vi "MartinsDCposition.vi"() -> ()   [LabVIEW 2011]
uses:
  Sub VIs/Trap cluster.ctl
  <vilib>/Utility/inputDevices.llb/closeKeyboard.vi
  <vilib>/Utility/inputDevices.llb/keyboardAcquire.vi
  <vilib>/vision/driver/NI_Vision_Acquisition_Software.lvlib
panel:
  in  "e_desired":sgl=0.5
  in  "Apply Corrections":bool
  in  "View Licence":bool
  in  "ok":bool caption="Mark the center of \nthe spot using the \nzoom and the point\ntool, then click this \nbutton"
  in  "Stop program":bool
  in  "Updating trap cluster":bool
  out "Camera enabled":bool
  out "SLM enabled":bool
  in  "Run calibration":bool
  in  "Hologram generation":cluster{"Method":i32, "Iterations":i32}={"Method"=0, "Iterations"=10} {"Method" items=["Lenses & Gratings (3D)", " Gerchberg-Saxton (3D)", "Gerchberg-Saxton FFT (2D)"]}
  in  "Display hologram\nand computed \nimage plane":bool=TRUE
  in  "ROI":T1={"Global Rectangle"=[568, 568, 719, 569], "Contours"=[{"Contour Type"=0, "ROI Type"=1, "Points"=[568, 568]}, {"Contour Type"=0, "ROI Type"=1, "Points"=[642, 568]}, {"Contour Type"=0, "ROI Type"=1, "Points"=[718, 568]}]}
  out "Image":T2(plugin-control)
  in  "y":dbl=100.0 min=1e-22
  in  "Show image":bool=TRUE
  in  "ROI size":dbl=2.0 min=2.0 step=2.0
  in  "Tab Control":enum32{"Normal", "Grid"}(tab)=enum."Grid"
  in  "Z":dbl[](array[numeric])=[0.0, 0.0, 0.0]
  in  "I":dbl[](array[numeric])=[10.0, 10.0, 10.0]
  out "#":i32[](array[numeric])=[0, 1, 2]
  in  "G":bool[](array[boolean])=[FALSE, FALSE, FALSE]
  in  "Spots y":i32=3
  in  "Grid spacing":i32=35
  in  "Spots x":i32=3
  in  "separation step":i32=1
  in  "max separation":i32=40
  in  "min separation":i32=30
  in  "Measure":bool
  in  "#images":i32=1
  out "Step number":i32
  in  "Move one spot":bool
  out "Calculated image plane":dbl[][](graph)
  out "Current trap pos":T3={"X (IMAQ)"=[555.0, 642.5, 730.0, 555.0, 642.5, 730.0, 555.0, 642.5, 730.0], "Y (IMAQ)"=[555.0, 555.0, 555.0, 642.5, 642.5, 642.5, 730.0, 730.0, 730.0], "Z"=[0.0, 0.0, 0.0, 0.0, 0.0, 0.0, 0.0, 0.0, 0.0], "Amplitudes"=[1.0, 1.0, 1.0, 1.0, 1.0, 1.0, 1.0, 1.0, 1.0], "Trap number"=[0, 1, 2, 3, 4, 5, 6, 7, 8], "ROI number"=[0, 1, 2, 3, 4, 5, 6, 7, 8], "Number of traps"=9, "Group"=[FALSE, FALSE, FALSE, FALSE, FALSE, FALSE, FALSE, FALSE, FALSE]}
  out "NI Vision error":errorcluster
  out "CUDA/SLM error":errorcluster
  in  "Cancel calibration":bool
  in  "Skip step if \ntimed out":bool
  in  "Display path":bool=TRUE
  out "Average step time (ms)":dbl
  in  "Step time \n(ms)":u32=10
  in  "Pause":bool
  in  "cancel path":bool
  out "Step skipped":bool
  in  "Path controls":T4={"follow path"=FALSE, "Step length"=1.0, "Arrive \nsimultaneously"=TRUE, "Synchronize traps"=FALSE, "Add current \npositions to path"=FALSE}
  in  "Create path":bool
  in  "Positioning  mode":enum16{"Normal", "Group", "Grid"}(ring)=enum."Grid"
  in  "Move \nHandle":bool
  out "Displayed Hologram":u8[][](graph)
  in  "Coordinate mapping \n(IMAQ to SLM)":T5={"sX"=-256.0, "sY"=-256.0, "sZ"=0.0, "cX"=0.4, "cY"=0.4, "cZ"=1.0}
  in  "Switch X/Y":bool
  # "Martin\nPersson 2011"
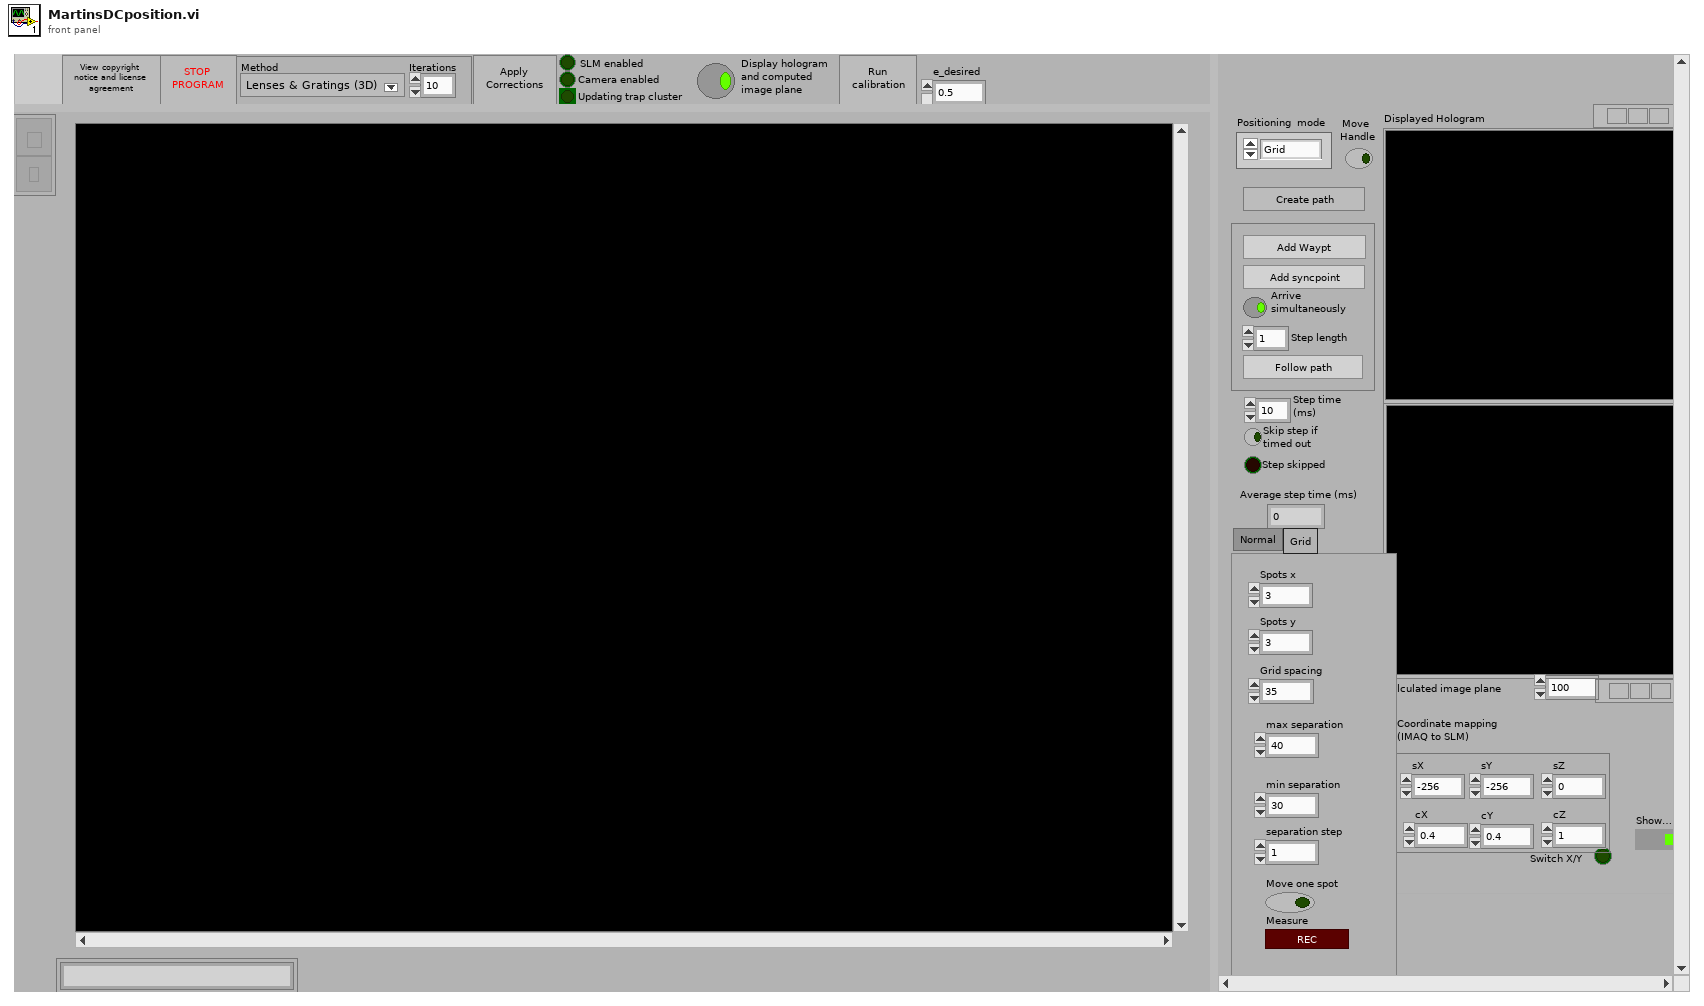
[diagram p1: front panel]
types:
  T1 = cluster{"Global Rectangle":i32[], "Contours":cluster{"Contour Type":u32, "ROI Type":u32, "Points":i32[]}[]}
  T2 = typedef "IMAQ Image.ctl" = refnum<image>
  T3 = typedef "Trap cluster.ctl" = cluster{"X (IMAQ)":dbl[], "Y (IMAQ)":dbl[], "Z":dbl[], "Amplitudes":dbl[], "Trap number":i32[], "ROI number":i32[], "Number of traps":i32, "Group":bool[]}
  T4 = cluster{"follow path":bool, "Step length":dbl, "Arrive \nsimultaneously":bool, "Synchronize traps":bool, "Add current \npositions to path":bool}
  T5 = cluster{"sX":dbl, "sY":dbl, "sZ":dbl, "cX":dbl, "cY":dbl, "cZ":dbl}
  T6 = cluster{"Centroid X":dbl[], "Centroid Y":dbl[], "Acquired Buffer Number":u32}
  T7 = typedef "IMAQdx.ctl" = refnum<k21>
  T8 = typedef "Image Type" = u32
  T9 = typedef "Semaphore RefNum" = refnum<k1>
  T10 = enum16{"0", "1", "2", "3", "4", "5", "6", "7", "8", "9", "A", "B", "C", "D", "E", "F", "G", "H", "I", "J", "K", "L", "M", "N", "O", "P", "Q", "R", "S", "T", "U", "V", "W", "X", "Y", "Z", "F1", "F2", "F3", "F4", "F5", "F6", "F7", "F8", "F9", "F10", "F11", "F12", "F13", "F14", "F15", "ADD", "BACK", "BACKSLASH", "CAPITAL", "COMMA", "DECIMAL", "DELETE", "DIVIDE", "DOWN", "END", "EQUALS", "ESCAPE", "GRAVE (`)", "HOME", "INSERT", "LBRACKET", "LCONTROL", "LEFT", "L ALT", "LSHIFT", "LWIN", "MINUS", "MULTIPLY", "NEXT", "NUMLOCK", "NUMPAD_0", "NUMPAD_1", "NUMPAD_2", "NUMPAD_3", "NUMPAD_4", "NUMPAD_5", "NUMPAD_6", "NUMPAD_7", "NUMPAD_8", "NUMPAD_9", "PAUSE", "PERIOD", "PRIOR (PG UP)", "RBRACKET", "RCONTROL", "RETURN", "RIGHT", "R ALT", "RSHIFT", "RWIN", "SCROLL", "SEMICOLON", "SLASH", "SPACE", "SUBTRACT", "TAB", "UP", "ENTER (num pad)", "' (quote)"}[]
  T11 = typedef "LVRectTypeDef.ctl" = cluster{"left":i16, "top":i16, "right":i16, "bottom":i16}
  T12 = cluster{"Contour Type":u32, "ROI Type":u32, "Points":i32[]}[]
  T13 = cluster{"Contour Type":u32, "ROI Type":u32, "Points":i32[]}
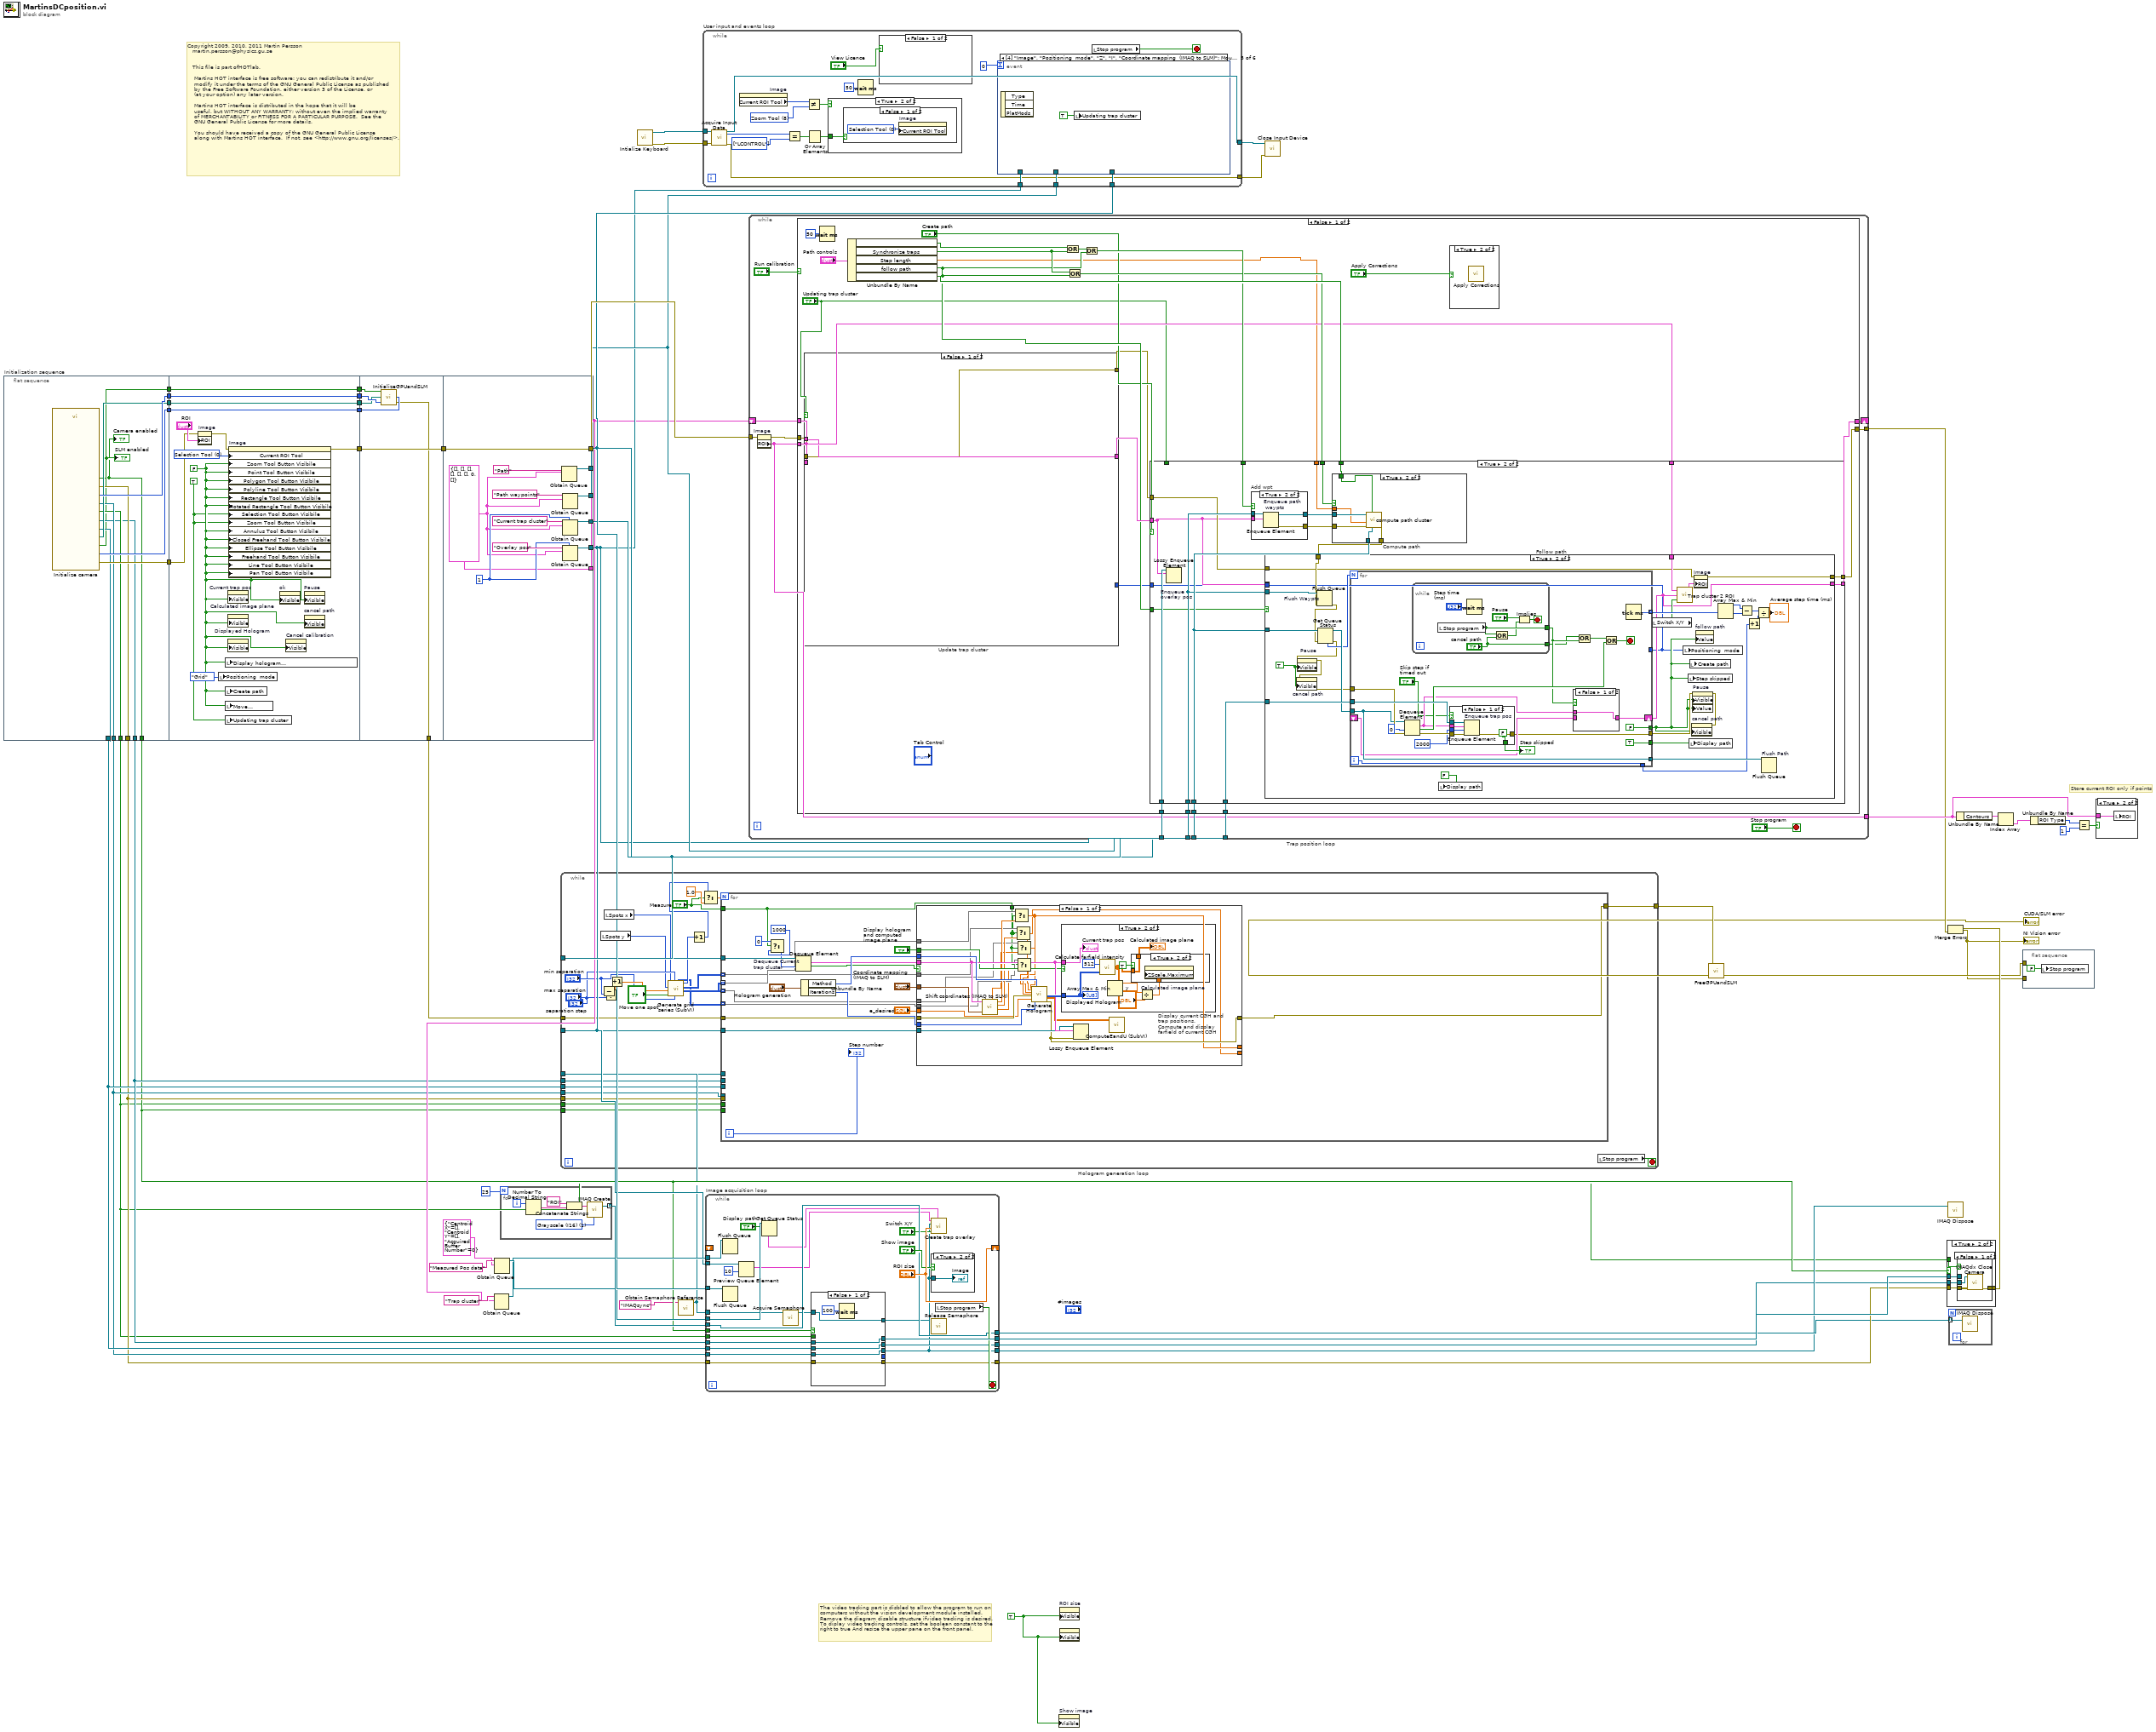
[diagram p0: block diagram]
diagram:
  w41 = TRUE ("Visible")
  # "Copyright 2009, 2010, 2011 Martin Persson \n   martin.persson@physics.gu.se\n\n\n   This file is part ofHOTlab.\n\n    Martins HOT interface is free software: you can redistribute it and/or \n    modify it under the terms of the GNU General Public License as published \n    by the Free Software Foundation, either version 3 of the License, or\n    (at your option) any later version.\n\n    Martins HOT interface is distributed in the hope that it will be \n    useful, but WITHOUT ANY WARRANTY; without even the implied warranty\n    of MERCHANTABILITY or FITNESS FOR A PARTICULAR PURPOSE.  See the\n    GNU General Public License for more details.\n\n    You should have received a copy of the GNU General Public License\n    along with Martins HOT interface.  If not, see <http://www.gnu.org/licenses/>."
  # "Store current ROI only if points"
  # "The video tracking part is disbled to allow the program to run on\ncomputers without the vision development module installed. \nRemove the diagram disable structure ifvideo tracking is desired. \nTo diplay video tracking controls, set the boolean constant to the \nright to true And resize the upper pane on the front panel."
  n1 = flat-sequence "Initialization sequence" {
    tunnel: [w56] -> w26
    tunnel: [w65] -> w25
    tunnel: [w64] -> w24
    tunnel: [w63] -> w23
    tunnel: [w62] -> w22
    tunnel: [w61] -> w6
    tunnel: [w60] -> w7
    tunnel: [w59] -> w5
    tunnel: [w58] -> w3
    tunnel: [w57] -> w8
    tunnel: [w55] -> w4
    tunnel: w26 -> [w74]
    tunnel: w25 -> [w72]
    tunnel: w24 -> [w77]
    tunnel: w23 -> [w76]
    tunnel: w22 -> [w75]
    tunnel: [w74] -> w15
    tunnel: [w67] -> w14
    tunnel: [w77] -> w12
    tunnel: [w76] -> w11
    tunnel: [w75] -> w10
    tunnel: w15 -> [w80]
    tunnel: w14 -> [w83]
    tunnel: [w83] -> w13
    tunnel: w12 -> [w81]
    tunnel: w11 -> [w82]
    tunnel: w10 -> [w79]
    tunnel: [w78] -> w9
    tunnel: [w94] -> w21
    tunnel: w13 -> [w94]
    tunnel: [w92] -> w20
    tunnel: [w90] -> w19
    tunnel: [w88] -> w18
    tunnel: [w87] -> w17
    tunnel: [w84] -> w16
    frame #0 {
      n2 = call "Initialize camera.vi"() -> ("CUDA device ID"=w63:i32, "IMAQdx Session Out"=w60:T7, "TrueFrame out"=w64:i32, "IMAQ camera"=w58:bool, "Image reference out"=w61:T2, "SLM enabled"=w56:bool, "Camera enabled"=w55:bool, "Vision error out"=w65:errorcluster, "LUT path out"=w62:path, "IMAQ Session Out"=w57:refnum<k11>, "Camera error"=w59:errorcluster)  [unwired: 5 in]
      "Camera enabled" <- w55
      "SLM enabled" <- w56
    }
    frame #1 {
      w70 = TRUE ("ROI Tool Buttons Visibile:Zoom Tool Button Visible")
      w71 = FALSE ("ROI Tool Buttons Visibile:Zoom Tool Button Visible")
      w69 = u32 0 items=["Zoom Tool"=8, "Selection Tool"=0, "Pan Tool"=9, "Point Tool"=1, "Line Tool"=2, "Rectangle Tool"=3, "Rotated Rectangle Tool"=12, "Polyline Tool"=10, "Polygon Tool"=5, "Freehand Tool"=11, "Closed Freehand Tool"=6, "Ellipse Tool"=4, "Annulus Tool"=7] ("Current ROI Tool")
      n3 = property on="Image" class="ImageControl"(error in=w72, "ROI"="ROI") -> (error out=w68:errorcluster)  [unwired: 1 in, 1 out]
      n4 = local write "Positioning  mode"(enum16{"Normal", "Group", "Grid"}."Grid" ("Positioning  mode")) -> ()
      n5 = local write "Display hologram\nand computed \nimage plane"(w71) -> ()
      n6 = local write "Create path"(w71) -> ()
      n7 = local write "Move \nHandle"(w71) -> ()
      n8 = local write "Updating trap cluster"(w70) -> ()
      n9 = property on="Current trap pos" class="Clust (strict)"("Visible"=w71) -> ()  [unwired: 2 in, 2 out]
      n10 = property on="Calculated image plane" class="IntGraph (strict)"("Visible"=w71) -> ()  [unwired: 2 in, 2 out]
      n11 = property on="Displayed Hologram" class="IntGraph (strict)"("Visible"=w71) -> ()  [unwired: 2 in, 2 out]
      n12 = property on="Image" class="ImageControl"(error in=w68, "Current ROI Tool"=w69, "Zoom Tool Button Visibile"=w71, "Point Tool Button Visibile"=w71, "Polygon Tool Button Visibile"=w71, "Polyline Tool Button Visibile"=w71, "Rectangle Tool Button Visibile"=w71, "Rotated Rectangle Tool Button Visibile"=w71, "Selection Tool Button Visibile"=w70, "Zoom Tool Button Visibile"=w70, "Annulus Tool Button Visibile"=w71, "Closed Freehand Tool Button Visibile"=w71, "Ellipse Tool Button Visibile"=w71, "Freehand Tool Button Visibile"=w71, "Line Tool Button Visibile"=w71, "Pan Tool Button Visibile"=w71) -> (error out=w67:errorcluster)  [unwired: 1 in, 1 out]
      n13 = property on="ok" class="Bool"("Visible"=w71) -> ()  [unwired: 2 in, 2 out]
      n14 = property on="Cancel calibration" class="Bool"("Visible"=w71) -> ()  [unwired: 2 in, 2 out]
      n15 = property on="Pause" class="Bool (strict)"("Visible"=w71) -> ()  [unwired: 2 in, 2 out]
      n16 = property on="cancel path" class="Bool"("Visible"=w71) -> ()  [unwired: 2 in, 2 out]
    }
    frame #2 {
      n17 = call "InitializeGPUandSLM.vi"("TrueFrame"=w81, "deviceId"=w82, "Path to LUT file"=w79, "SLM enabled"=w80) -> ("CUDA/SLM error"=w78:errorcluster)  [unwired: 1 out]
    }
    frame #3 {
      w85 = 1 ("max queue size (-1, unlimited)")
      w84 = T3 {"X (IMAQ)"=[], "Y (IMAQ)"=[], "Z"=[], "Amplitudes"=[], "Trap number"=[], "ROI number"=[], "Number of traps"=0, "Group"=[]} ("output cluster 2")
      n18 = Obtain Queue(name (unnamed)="Path", element data type=w84) -> (queue out=w92:refnum<queue>)  [unwired: 3 in, 2 out]
      n19 = Obtain Queue(name (unnamed)="Path waypoints", element data type=w84) -> (queue out=w90:refnum<queue>)  [unwired: 3 in, 2 out]
      n20 = Obtain Queue(max queue size (-1, unlimited)=w85, name (unnamed)="Current trap cluster", element data type=w84) -> (queue out=w88:refnum<queue>)  [unwired: 2 in, 2 out]
      n21 = Obtain Queue(max queue size (-1, unlimited)=w85, name (unnamed)="Overlay pos", element data type=w84) -> (queue out=w87:refnum<queue>)  [unwired: 2 in, 2 out]
    }
  }
  n22 = Obtain Queue(name (unnamed)="Trap cluster", element data type=w16) -> (queue out=w46:refnum<queue>)  [unwired: 3 in, 2 out]
  n23 = Obtain Queue(name (unnamed)="Measured Pos data", element data type=T6 {"Centroid X"=[], "Centroid Y"=[], "Acquired Buffer Number"=0} ("output cluster 2")) -> (queue out=w49:refnum<queue>)  [unwired: 3 in, 2 out]
  n24 = for {
    N: 25 -> [_]
    tunnel: [w100] -> w51 mode=indexing
    i -> [w96]
    w98 = T8 1 items=["Grayscale (U8)", "Grayscale (I16)", "Grayscale (SGL)", "Complex (CSG)", "RGB (U32)", "HSL (U32)", "RGB (U64)", "Grayscale (U16)"] ("Image Type")
    n25 = Number To Decimal String(number=w96) -> (decimal integer string=w95:string)  [unwired: 1 in]
    n26 = Concatenate Strings("ROI" ("Image Name"), w95) -> (w97:string)
    n27 = call "IMAQ Create"("Image Name"=w97, "Image Type"=w98) -> ("New Image"=w100:T2)  [unwired: 3 in, 1 out]
  }
  n28 = call <vilib>:"Intialize Keyboard.vi"() -> ("error out"=w28:errorcluster, "device ID"=w54:refnum<k1>)  [unwired: 1 in, 9 out]
  n29 = call <vilib>:"Obtain Semaphore Reference.vi"("name (unnamed)"="IMAQsync") -> ("semaphore"=w1:T9)  [unwired: 4 in, 2 out]
  n30 = while "Hologram generation loop" {
    tunnel: w18 -> [w129]
    tunnel: w17 -> [w127]
    tunnel: w9 -> [w128]
    tunnel: [w122] -> w32
    tunnel: w8 -> [w126]
    tunnel: w7 -> [w125]
    tunnel: w6 -> [w124]
    tunnel: w5 -> [w123]
    tunnel: w4 -> [w121]
    tunnel: w3 -> [w120]
    tunnel: w1 -> [w119]
    stop <- w130 stop-if-true
    n31 = local read "Spots y"() -> (w108:i32)
    n32 = Subtract(x="max separation", y="min separation") -> (x-y=w114:i32)
    n33 = Divide(x=w114, y="separation step") -> (x/y=w113:dbl)
    n34 = local read "Spots x"() -> (w109:i32)
    n35 = Increment(x=w113) -> (x+1=w112:dbl)
    n36 = call "Generate grid series (SubVI).vi"("min separation"="min separation", "separation step"="separation step", "Move one spot"="Move one spot", "Number of steps"=w112, "Spots y"=w108, "Spots x"=w109) -> ("Array 2"=w105:i32[][], "Array"=w104:i32[][], "Numeric out"=w107:i32, "Z"=w103:i32[][], "A"=w102:i32[][])  [unwired: 1 in]
    n37 = Increment(x=w107) -> (x+1=w106:i32)
    n38 = Select(t=w106, s="Measure", f=1.0) -> (s? t:f=w118:dbl)
    n39 = for {
      N: w118 -> [_]
      tunnel: w129 -> [w149]
      tunnel: w128 -> [w144]
      tunnel: w127 -> [w142]
      tunnel: w126 -> [_]
      tunnel: w125 -> [_]
      tunnel: w124 -> [_]
      tunnel: w123 -> [_]
      tunnel: [w131] -> w122
      tunnel: w121 -> [_]
      tunnel: w120 -> [_]
      tunnel: w119 -> [_]
      tunnel: "Measure" -> [w133]
      tunnel: w105 -> [w137] mode=indexing
      tunnel: w104 -> [w136] mode=indexing
      tunnel: w103 -> [w135] mode=indexing
      tunnel: w102 -> [w134] mode=indexing
      i -> [w132]
      n40 = Select(t=0, s=w133, f=1000 ("timeout in ms (-1)")) -> (s? t:f=w138:i32)
      n41 = Dequeue Element "Dequeue Current \ntrap cluster"(queue=w149, timeout in ms (-1)=w138) -> (element=w148:T3, timed out?=w141:bool)  [unwired: 1 in, 2 out]
      n42 = Unbundle By Name("Hologram generation") -> ("Method"=w151:i32, "Iterations"=w150:i32)
      n43 = case shown="False" w141 {
        tunnel: "Coordinate mapping \n(IMAQ to SLM)" -> [w175 _]
        tunnel: "Display hologram\nand computed \nimage plane" -> [w169 _]
        tunnel: w151 -> [w173 _]
        tunnel: w150 -> [w172 _]
        tunnel: w148 -> [w171 _]
        tunnel: w142 -> [w170 _]
        tunnel: w144 -> [w168 w187]
        tunnel: [w166 w187] -> w131
        tunnel: "e_desired" -> [w167 _]
        tunnel: [w154 _] -> _
        tunnel: [w153 _] -> _
        tunnel: w137 -> [w163 _]
        tunnel: w136 -> [w162 _]
        tunnel: w135 -> [w161 _]
        tunnel: w134 -> [w160 _]
        tunnel: w133 -> [w155 _]
        frame False {
          n44 = call "Shift coordinates (IMAQ to SLM).vi"("Trap cluster"=w171, "Coordinate mapping \n(IMAQ to SLM)"=w175) -> ("X (SLM)"=w165:sgl[], "Y (SLM)"=w164:sgl[], "Intensities"=w158:sgl[], "Z (SLM)"=w157:sgl[])  [unwired: 1 in, 1 out]
          n45 = Select(t=w163, s=w155, f=w165) -> (s? t:f=w154:sgl[])
          n46 = Select(t=w162, s=w155, f=w164) -> (s? t:f=w153:sgl[])
          n47 = Select(t=w161, s=w155, f=w157) -> (s? t:f=w156:sgl[])
          n48 = Select(t=w160, s=w155, f=w158) -> (s? t:f=w159:sgl[])
          n49 = call "Generate Hologram.vi"("x"=w154, "y"=w153, "z"=w156, "spot_intensities"=w159, "CUDA/SLM error in"=w168, "e_desired"=w167, "N_iterations"=w172, "method"=w173) -> ("CGH out"=w174:u8[][], "weights"=w152:sgl[][], "CUDA/SLM error out"=w166:errorcluster)  [unwired: 16 in, 1 out]
          n50 = case "Display current CGH and trap positions.\nCompute and display farfield of current CGH" shown="True" w169 {
            tunnel: w174 -> [_ w184]
            tunnel: w171 -> [_ w183]
            frame False {
            }
            frame True {
              n51 = call "Calculate farfield intensity.vi"("h_pSLM"=w184, "Numeric"=512) -> ("Calculated image plane"=w178:dbl[][])
              n52 = Array Max & Min(array=w178) -> (max value=w181:dbl)  [unwired: 3 out]
              n53 = Divide(x=w181, y="y") -> (x/y=w179:dbl)
              n54 = case shown="True" TRUE {
                tunnel: w179 -> [_ w186]
                tunnel: w178 -> [_ w185]
                tunnel: [_ w185] -> w177
                frame False {
                }
                frame True {
                  n55 = property on="Calculated image plane" class="IntGraph (strict)"("ZScale.Maximum"=w186) -> ()  [unwired: 2 in, 2 out]
                }
              }
              "Calculated image plane" <- w177
              "Displayed Hologram" <- w184
              "Current trap pos" <- w183
            }
          }
          n56 = Lossy Enqueue Element(queue=w170, element=w171, error in (no error)=w166) -> ()  [unwired: 4 out]
          n57 = call "ComputeEandU (SubVI).vi"("weights in"=w152) -> ()  [unwired: 9 in, 2 out]
        }
        frame True {
        }
      }
      "Step number" <- w132
    }
    n58 = local read "Stop program"() -> (w130:bool)
  }
  n59 = while "User input and events loop" {
    tunnel: w54 -> [w205]
    tunnel: w17 -> [w194]
    tunnel: w19 -> [w193]
    tunnel: w20 -> [w192]
    tunnel: [w191] -> w29
    tunnel: w28 -> [w190]
    tunnel: [w189] -> w27
    stop <- w197 stop-if-true
    w202 = u32 8 items=["Zoom Tool"=8, "Selection Tool"=0, "Pan Tool"=9, "Point Tool"=1, "Line Tool"=2, "Rectangle Tool"=3, "Rotated Rectangle Tool"=12, "Polyline Tool"=10, "Polygon Tool"=5, "Freehand Tool"=11, "Closed Freehand Tool"=6, "Ellipse Tool"=4, "Annulus Tool"=7] ("Current ROI Tool")
    w199 = T10 [enum."LCONTROL"] items=["0", "1", "2", "3", "4", "5", "6", "7", "8", "9", "A", "B", "C", "D", "E", "F", "G", "H", "I", "J", "K", "L", "M", "N", "O", "P", "Q", "R", "S", "T", "U", "V", "W", "X", "Y", "Z", "F1", "F2", "F3", "F4", "F5", "F6", "F7", "F8", "F9", "F10", "F11", "F12", "F13", "F14", "F15", "ADD", "BACK", "BACKSLASH", "CAPITAL", "COMMA", "DECIMAL", "DELETE", "DIVIDE", "DOWN", "END", "EQUALS", "ESCAPE", "GRAVE (`)", "HOME", "INSERT", "LBRACKET", "LCONTROL", "LEFT", "L ALT", "LSHIFT", "LWIN", "MINUS", "MULTIPLY", "NEXT", "NUMLOCK", "NUMPAD_0", "NUMPAD_1", "NUMPAD_2", "NUMPAD_3", "NUMPAD_4", "NUMPAD_5", "NUMPAD_6", "NUMPAD_7", "NUMPAD_8", "NUMPAD_9", "PAUSE", "PERIOD", "PRIOR (PG UP)", "RBRACKET", "RCONTROL", "RETURN", "RIGHT", "R ALT", "RSHIFT", "RWIN", "SCROLL", "SEMICOLON", "SLASH", "SPACE", "SUBTRACT", "TAB", "UP", "ENTER (num pad)", "' (quote)"] ("keys pressed")
    n60 = call-poly <vilib>:"Acquire Input Data.vi"("device ID"=w205, "error in (no error)"=w190) -> ("device ID"=w191:refnum<k1>, "keys pressed"=w198:T10, "error out"=w189:errorcluster)  [unwired: 15 out]
    n61 = property on="Image" class="ImageControl"() -> ("Current ROI Tool"=w201:u32)  [unwired: 2 in, 2 out]
    n62 = Equal?(x=w198, y=w199) -> (x = y?=w200:bool[])
    n63 = Not Equal?(x=w201, y=w202) -> (x != y?=w203:bool)
    n64 = Or Array Elements(Boolean array=w200) -> (logical OR=w204:bool)
    n65 = case shown="True" w203 {
      tunnel: w204 -> [_ w226]
      frame False {
      }
      frame True {
        n66 = case shown="False" w226 {
          frame False {
            w227 = u32 0 items=["Zoom Tool"=8, "Selection Tool"=0, "Pan Tool"=9, "Point Tool"=1, "Line Tool"=2, "Rectangle Tool"=3, "Rotated Rectangle Tool"=12, "Polyline Tool"=10, "Polygon Tool"=5, "Freehand Tool"=11, "Closed Freehand Tool"=6, "Ellipse Tool"=4, "Annulus Tool"=7] ("Current ROI Tool")
            n67 = property on="Image" class="ImageControl"("Current ROI Tool"=w227) -> ()  [unwired: 2 in, 2 out]
          }
          frame True {
            w228 = u32 1 items=["Zoom Tool"=8, "Selection Tool"=0, "Pan Tool"=9, "Point Tool"=1, "Line Tool"=2, "Rectangle Tool"=3, "Rotated Rectangle Tool"=12, "Polyline Tool"=10, "Polygon Tool"=5, "Freehand Tool"=11, "Closed Freehand Tool"=6, "Ellipse Tool"=4, "Annulus Tool"=7] ("Current ROI Tool")
            n68 = property on="Image" class="ImageControl"("Current ROI Tool"=w228) -> ()  [unwired: 2 in, 2 out]
          }
        }
      }
    }
    n69 = Wait (ms)(milliseconds to wait=u32 50) -> ()  [unwired: 1 out]
    n70 = case shown="False" "View Licence" {
      frame False {
      }
      frame True {
        n71 = call "View license.vi"() -> ()  [unwired: 1 in]
      }
    }
    n72 = event shown="[4] \"Image\", \"Positioning  mode\", \"Z\", \"I\", \"Coordinate mapping \n(IMAQ to SLM)\": Mouse Down;  Key Up" {
      selector: _ -> [_ _ _ _ _ _]
      dyn-events: _ -> [_ _ _ _ _ _]
      timeout: 0 -> [_ _ _ _ _ _]
      tunnel: w194 -> [_ _ w216 _ _ _]
      tunnel: w193 -> [_ _ w215 _ _ _]
      tunnel: w192 -> [_ _ w219 _ _ _]
      event Timeout {
        n73 = event-data() -> ()  [unwired: 1 in, 2 out]
      }
      event "Display hologram\nand computed \nimage plane": Value Change {
        n74 = event-data() -> ("NewVal"=w207:bool)  [unwired: 1 in, 4 out]
        n75 = property on="Current trap pos" class="Clust (strict)"("Visible"=w207) -> ()  [unwired: 2 in, 2 out]
        n76 = property on="Displayed Hologram" class="IntGraph (strict)"("Visible"=w207) -> ()  [unwired: 2 in, 2 out]
        n77 = property on="Calculated image plane" class="IntGraph (strict)"("Visible"=w207) -> ()  [unwired: 2 in, 2 out]
        n78 = property on="Property Node" class="VI"() -> ("Front Panel.WinBounds"=w214:T11)  [unwired: 2 in, 2 out]
        n79 = Unbundle By Name(w214) -> ("right"=w213:i16, "left"=w212:i16)
        n80 = Subtract(x=w213, y=w212) -> (x-y=w211:i16)
        n81 = Select(t=i16 500 ("x-y"), s=w207, f=i16 196 ("x-y")) -> (s? t:f=w206:i16)
        n82 = Subtract(x=w211, y=w206) -> (x-y=w210:i16)
        n83 = property on="Splitter" class="Splitter"("Position"=w210) -> ()  [unwired: 2 in, 2 out]